vi "UHR-Fleezers Control (host) - 10.8MV_trial.vi"() -> ()   [LabVIEW 2010] (continued)
      n270 = call <vilib>:"Application Directory.vi"() -> ("Application Directory"=w928:path)
      n271 = Build Path(base path=w928, name or relative path="_trap_screen_positions") -> (appended path=w936:path)
      n272 = Open/Create/Replace File(file path (use dialog)=w936, operation (0:open)=T25."open or create", access (0:read/write)=enum16{"read/write", "read-only", "write-only"}."read/write") -> (refnum out=w938:refnum<file>)  [unwired: 3 in, 2 out]
      n273 = local read "Trap Sets"() -> (w930:u32)
      n274 = for "Load trap positions on video screen from file." {
        N: w930 -> [_]
        tunnel: [w956] -> w931
        tunnel: w938 -> [w955]
        tunnel: [w952] -> w927 mode=indexing
        w954 = 4
        n275 = for {
          N: w954 -> [_]
          tunnel: [w960] -> w956
          tunnel: w955 -> [w959]
          tunnel: w954 -> [w958]
          tunnel: [w957] -> w953 mode=indexing
          n276 = Read from Binary File(5:w958, 11:w959) -> (2:w957:i32, 3:w960:refnum<file>)  [unwired: 4 in, 2 out]
        }
        n277 = Array To Cluster(array=w953) -> (cluster=w952:T29)
      }
      n278 = node-c288() -> (w951:T26)  [unwired: 4 in]
      n279 = timed-loop "acquire video and stage position" {
        timing: w951 -> [_]
        timing-out: [_] -> w950
        tunnel: w943 -> [w979]
        tunnel: w942 -> [w978]
        tunnel: w941 -> [w977]
        tunnel: [w976] -> w923
        tunnel: [w973] -> w924
        tunnel: [w974] -> w922
        tunnel: w949 -> [_]
        shift-right: [w970] -> w940
        shift-left: w927 -> [w971]
        tunnel: w930 -> [w968]
        stop <- w975 stop-if-true
        n280 = node-c288() -> ()  [unwired: 1 in, 1 out]
        n281 = event shown="[2] \"Primary Video Display\": Mouse Down" {
          selector: _ -> [_ _ _ _]
          dyn-events: _ -> [_ _ _ _]
          timeout: 10 -> [_ _ _ _]
          tunnel: w979 -> [w990 w1005 w1014 w1033]
          tunnel: w978 -> [w989 w1007 w1012 w1035]
          tunnel: w977 -> [w988 w1006 w1013 w1034]
          tunnel: [w987 w1005 w1014 w1033] -> w976
          tunnel: [w980 w1009 FALSE FALSE] -> w975
          tunnel: [w984 w1007 w1012 w1035] -> w974
          tunnel: [w983 w1006 w1013 w1034] -> w973
          tunnel: "radius" -> [_ _ w1019 _]
          tunnel: w971 -> [w981 w1008 w1017 _]
          tunnel: [w981 w1008 w1018 cluster{i32, i32, i32, i32}[] []] -> w970
          tunnel: w968 -> [_ _ w1010 _]
          event Timeout {
            n282 = event-data() -> ()  [unwired: 1 in, 2 out]
            n283 = call <vilib>:"IMAQ Grab Acquire.vi"("error in (no error)"=w989, "Image In"=w988, "IMAQ Session In"=w990) -> ("error out"=w985:errorcluster, "Image Out"=w986:T2, "IMAQ Session Out"=w987:refnum<k11>)  [unwired: 5 in, 1 out]
            n284 = case shown="True" "trap\nmarkers?" {
              tunnel: w981 -> [_ w998]
              tunnel: w986 -> [w992 w997]
              tunnel: w985 -> [w991 w996]
              tunnel: [w991 w995] -> w984
              tunnel: [w992 w993] -> w983
              frame False {
              }
              frame True {
                n285 = for {
                  tunnel: w998 -> [w1004] mode=indexing
                  shift-right: [w1002] -> w993
                  shift-left: w997 -> [w1003]
                  tunnel: w996 -> [w1001]
                  tunnel: [w1000] -> w995
                  tunnel: u32 16711680 ("Color") -> [w999]
                  n286 = call "IMAQ Overlay Oval"("Color"=w999, "error in (no error)"=w1001, "Bounding Rectangle"=w1004, "Image"=w1003) -> ("error out"=w1000:errorcluster, "Image Out"=w1002:T2)  [unwired: 6 in]
                }
              }
            }
            "Primary Video Display" <- w983
            n287 = Unbundle By Name(w985) -> ("status"=w980:bool)
          }
          event "Stop All": Value Change {
            n288 = event-data() -> ()  [unwired: 1 in, 5 out]
            n289 = local read "Stop All"() -> (w1009:bool)
          }
          event "Primary Video Display": Mouse Down {
            n290 = event-data() -> ()  [unwired: 1 in, 7 out]
            n291 = Array Size(array=w1017) -> (size(s)=w1016:i32)
            n292 = Less?(x=w1016, y=w1010) -> (x < y?=w1015:bool)
            n293 = case shown="True" w1015 {
              tunnel: w1019 -> [_ w1029]
              tunnel: w1017 -> [w1020 w1023]
              tunnel: [w1020 w1022] -> w1018
              frame False {
              }
              frame True {
                n294 = property on="Primary Video Display" class="ImageControl"() -> ("Last Mouse Position"=w1021:cluster{"X":i32, "Y":i32})  [unwired: 2 in, 2 out]
                n295 = Unbundle By Name(w1021) -> ("X"=w1031:i32, "Y"=w1030:i32)
                n296 = Add(x=w1030, y=w1029) -> (x+y=w1027:i32)
                n297 = Subtract(x=w1030, y=w1029) -> (x-y=w1025:i32)
                n298 = Add(x=w1031, y=w1029) -> (x+y=w1026:i32)
                n299 = Subtract(x=w1031, y=w1029) -> (x-y=w1028:i32)
                n300 = Bundle(w1028, w1027, w1026, w1025) -> (w1024:cluster{i32, i32, i32, i32})  [unwired: 1 in]
                n301 = Build Array (concatenate)(w1023, w1024) -> (w1022:T30)
              }
            }
          }
          event "clear markers": Value Change {
            n302 = event-data() -> ()  [unwired: 1 in, 5 out]
          }
        }
        n303 = node-c288() -> ()  [unwired: 1 in, 1 out]
      }
      n304 = node-c288(w950) -> ()  [unwired: 1 out]
      n305 = Set File Position(offset (in bytes) (0)=i64 0, refnum=w931, from (0:start)=enum16{"start", "end", "current"}."start") -> (refnum out=w932:refnum<file>)  [unwired: 1 in, 1 out]
      n306 = for "Write trap positions to file so they can be remembered\nwhen program is removed from memory" {
        tunnel: w940 -> [w964] mode=indexing
        tunnel: [w962] -> w939
        tunnel: w932 -> [w961]
        n307 = Cluster To Array(cluster=w964) -> (array=w963:i32[])
        n308 = for {
          tunnel: w963 -> [w967] mode=indexing
          tunnel: [w966] -> w962
          tunnel: w961 -> [w965]
          n309 = Write to Binary File(file (use dialog)=w965, data=w967) -> (refnum out=w966:refnum<file>)  [unwired: 4 in, 2 out]
        }
      }
      n310 = Close File(refnum=w939) -> ()  [unwired: 1 in, 2 out]
      n311 = call "IMAQ Dispose"("Image"=w924, "error in (no error)"=w922) -> ("error out"=w921:errorcluster)  [unwired: 4 in]
      n312 = call <vilib>:"IMAQ Stop.vi"("error in (no error)"=w921, "IMAQ Session In"=w923) -> ("error out"=w925:errorcluster, "IMAQ Session Out"=w926:refnum<k11>)  [unwired: 8 in]
      n313 = call <vilib>:"IMAQ Close.vi"("error in (no error)"=w925, "IMAQ Session In"=w926) -> ()  [unwired: 9 in, 1 out]
    }
    frame Enabled {
    }
  }
  n314 = node-c288(2 ("Processor")) -> (w15:T26)  [unwired: 3 in]
  n315 = node-c288() -> (w69:T26)  [unwired: 4 in]
  n316 = disable-structure shown="Enabled" {
    disable-tunnel: [w1042 _] -> w35
    disable-tunnel: w24 -> [w1041 _]
    frame Enabled {
      n317 = node-c288() -> (w1044:T26)  [unwired: 4 out]
      n318 = timed-loop "Rough control of MCL mirror stage (debugging)" {
        tunnel: w1041 -> [w1047]
        tunnel: [w1046] -> w1042
        timing: w1044 -> [_]
        timing-out: [_] -> w1043
        stop <- w1046 stop-if-true
        n319 = node-c288() -> ()  [unwired: 2 out]
        n320 = case shown="1" "MCL Mode" {
          tunnel: w1047 -> [_ w1050 w1154]
          frame 0, Default {
            # "manual positioning"
          }
          frame 1 {
            # "sinusoidal wave"
            n321 = node-c288() -> (w1052:T26)  [unwired: 4 out]
            n322 = timed-loop "Oscillate MCL mirror" {
              timing: w1052 -> [_]
              timing-out: [_] -> w1051
              tunnel: w1050 -> [w1091]
              i -> [w1090]
              stop <- w1053 stop-if-true
              n323 = node-c288() -> (w1089:i64)  [unwired: 1 out]
              n324 = Multiply(x="AO1", y=32767.0) -> (x*y=w1085:dbl)
              n325 = Multiply(x="AO2", y=32767.0) -> (x*y=w1080:dbl)
              n326 = Divide(x=w1085, y=10.0) -> (x/y=w1086:dbl)
              n327 = Divide(x=w1080, y=10.0) -> (x/y=w1081:dbl)
              n328 = To Word Integer(number=w1086) -> (16bit integer=w1078:i16)
              n329 = To Word Integer(number=w1081) -> (16bit integer=w1077:i16)
              n330 = Divide(x=w1089, y=i64 1000) -> (x/y=w1060:dbl)
              n331 = Multiply(x=w1060, y=w1090) -> (x*y=w1071:dbl)
              n332 = Multiply(x="Osc. freq. (Hz) 2", y=6.283185307179586) -> (x*y=w1072:dbl)
              n333 = Multiply(x=w1072, y=w1071) -> (x*y=w1070:dbl)
              n334 = Sine(x=w1070) -> (sin(x)=w1069:dbl)
              n335 = Multiply(x=w1069, y="Osc. amp. (V)") -> (x*y=w1067:dbl)
              n336 = Add(x=w1067, y="Osc. center (V)") -> (x+y=w1065:dbl)
              n337 = Divide(x=w1065, y=10.0) -> (x/y=w1063:dbl)
              n338 = Multiply(x=w1063, y=32767.0) -> (x*y=w1058:dbl)
              n339 = Select(t=w1058, s="Scan axis", f=w1078) -> (s? t:f=w1076:dbl)
              n340 = Select(t=w1077, s="Scan axis", f=w1058) -> (s? t:f=w1075:dbl)
              n341 = local read "MCL Mode"() -> (w1057:u16)
              n342 = Not Equal?(x=w1057, y=u16 1) -> (x != y?=w1054:bool)
              n343 = local read "Stop All"() -> (w1055:bool)
              n344 = xnode "Read/Write Control"("FPGA VI Reference In"=w1091, "AO1"=w1076, "AO2"=w1075) -> ()  [unwired: 1 in, 2 out]
              n345 = Compound Arithmetic op=OR(w1055, w1054) -> (w1053:bool)
              n346 = node-c288() -> ()  [unwired: 2 out]
            }
            n347 = node-c288(w1051) -> ()  [unwired: 1 out]
          }
          frame 2 {
            # "linear scan"
            n348 = case shown="True" "Start Scan" {
              tunnel: w1154 -> [_ w1166]
              frame False {
              }
              frame True {
                n349 = Subtract(x="End (V)", y="Begin (V)") -> (x-y=w1162:dbl)
                n350 = Decrement(x="N Points") -> (x-1=w1161:dbl)
                n351 = Divide(x=w1162, y=w1161) -> (x/y=w1159:dbl)
                n352 = for {
                  N: "N Points" -> [_]
                  tunnel: "Begin (V)" -> [w1179]
                  tunnel: w1166 -> [w1171]
                  tunnel: [w1170] -> w1165 mode=indexing
                  tunnel: w1159 -> [w1169]
                  tunnel: [w1167] -> w1158 mode=indexing
                  i -> [w1178]
                  n353 = Multiply(x=w1169, y=w1178) -> (x*y=w1177:dbl)
                  n354 = Add(x=w1179, y=w1177) -> (x+y=w1174:dbl)
                  n355 = local read "Scan axis"() -> (w1168:bool)
                  n356 = local read "AO1"() -> (w1176:dbl)
                  n357 = local read "AO2"() -> (w1175:dbl)
                  n358 = Select(t=w1174, s=w1168, f=w1176) -> (s? t:f=w1173:dbl)
                  n359 = Select(t=w1175, s=w1168, f=w1174) -> (s? t:f=w1172:dbl)
                  n360 = flat-sequence {
                    tunnel: w1173 -> [w1183]
                    tunnel: w1172 -> [w1182]
                    tunnel: w1171 -> [w1180]
                    tunnel: [w1250] -> w1170
                    tunnel: [w1249] -> w1167
                    frame #0 {
                      w1186 = 10.0 ("y")
                      w1181 = 32767.0 ("y")
                      n361 = Multiply(x=w1183, y=w1181) -> (x*y=w1189:dbl)
                      n362 = Multiply(x=w1182, y=w1181) -> (x*y=w1187:dbl)
                      n363 = Divide(x=w1189, y=w1186) -> (x/y=w1190:dbl)
                      n364 = Divide(x=w1187, y=w1186) -> (x/y=w1188:dbl)
                      n365 = To Word Integer(number=w1190) -> (16bit integer=w1184:i16)
                      n366 = To Word Integer(number=w1188) -> (16bit integer=w1185:i16)
                      n367 = xnode "Read/Write Control"("FPGA VI Reference In"=w1180, "AO1"=w1184, "AO2"=w1185) -> ()  [unwired: 1 in, 2 out]
                    }
                    frame #1 {
                      n368 = Wait (ms)(milliseconds to wait="DAQ Delay (ms)") -> ()  [unwired: 1 out]
                    }
                    frame #2 {
                      n369 = local read "Slow mean"() -> (w1250:dbl)
                      n370 = local read "Sigma"() -> (w1249:dbl)
                    }
                  }
                }
                n371 = Bundle("Begin (V)"="Begin (V)", w1159, w1165) -> (→"MCL Scan":cluster{"Begin (V)":dbl, dbl, dbl[]})  [unwired: 1 out]
                n372 = Bundle("Begin (V)"="Begin (V)", w1159, w1158) -> (→"MCL Scan 2":cluster{"Begin (V)":dbl, dbl, dbl[]})  [unwired: 1 out]
              }
            }
          }
        }
        n373 = local read "Stop All"() -> (w1046:bool)
        n374 = node-c288() -> ()  [unwired: 2 out]
      }
      n375 = node-c288(w1043) -> ()  [unwired: 1 out]
    }
    frame Disabled {
    }
  }
  n376 = timed-loop "Control parameters (event loop)" {
    tunnel: w24 -> [w1256]
    shift-right: [w1255] -> _
    shift-left: errorcluster {"status"=FALSE, "code"=0, "source"=""} ("error out") -> [w1254]
    tunnel: [w1253] -> w37
    timing: w15 -> [_]
    timing-out: [_] -> w14
    stop <- w1253 stop-if-true
    n377 = node-c288() -> ()  [unwired: 1 in, 1 out]
    n378 = event shown="[6] \"BD 1 Frequency 1 (MHz)\", \"BD 1 Frequency 2 (MHz)\", \"BD 1 Frequency 3 (MHz)\", \"BD 2 Frequency 1 (MHz)\", \"BD 2 Frequency 2 (MHz)\", \"BD 2 Frequency 3 (MHz)\", \"Trap Delta (MHz)\": Value Change" {
      selector: _ -> [_ _ _ _ _ _ _ _ _ _ _ _ _ _ _ _ _ _ _ _ _ _ _ _ _ _ _ _ _ _ _ _ _ _ _ _ _ _ _ _ _ _ _ _ _ _ _ _ _ _ _ _ _ _ _]
      dyn-events: _ -> [_ _ _ _ _ _ _ _ _ _ _ _ _ _ _ _ _ _ _ _ _ _ _ _ _ _ _ _ _ _ _ _ _ _ _ _ _ _ _ _ _ _ _ _ _ _ _ _ _ _ _ _ _ _ _]
      timeout: _ -> [_ _ _ _ _ _ _ _ _ _ _ _ _ _ _ _ _ _ _ _ _ _ _ _ _ _ _ _ _ _ _ _ _ _ _ _ _ _ _ _ _ _ _ _ _ _ _ _ _ _ _ _ _ _ _]
      tunnel: w1256 -> [w1294 _ _ _ w1416 _ w1513 _ w1577 _ _ _ w1772 _ _ w1874 w2018 w2082 w2157 w2311 w2388 w2519 w2615 w2701 w2787 w2873 w2959 w3045 w3138 w3302 w3513 _ w3658 w3795 _ w4002 w4044 w4092 w4171 w4213 _ w4259 _ _ _ _ w4450 _ w4543 w4584 w4631 w4819 w4868 _ w4930]
      tunnel: [w1293 _ _ _ w1406 _ w1512 _ w1540 _ w1737 _ w1751 _ _ w1873 w2014 w2079 w2154 w2310 w2386 w2518 w2609 w2695 w2781 w2867 w2953 w3039 w3136 w3301 w3511 _ w3656 w3793 _ w4000 w4042 w4082 w4169 w4211 _ w4257 _ _ _ _ w4448 _ _ _ _ _ _ _ _] -> w1255
      tunnel: w1254 -> [w1292 _ _ _ w1415 _ w1511 _ w1572 _ w1737 _ w1771 _ _ w1872 w2013 w2078 w2153 w2309 w2387 w2517 w2614 w2700 w2786 w2872 w2958 w3044 w3137 w3300 w3512 _ w3657 w3794 _ w4001 w4043 w4091 w4170 w4212 _ w4258 _ _ _ _ w4449 _ w4542 w4583 w4630 w4818 w4867 _ w4929]
      tunnel: [_ _ _ _ _ _ _ _ _ _ w1736 _ _ _ _ _ _ _ _ _ _ _ _ _ _ _ _ _ _ _ _ _ _ _ _ _ _ _ _ _ _ _ _ _ _ _ _ _ _ _ _ _ _ _ _] -> w1253
      tunnel: [_ _ _ _ _ _ _ "Round T1 X" _ _ _ _ _ _ _ _ _ _ _ _ _ _ _ _ _ _ _ _ _ _ _ _ _ _ _ _ _ _ _ _ _ _ _ _ _ _ _ _ _ _ _ _ _ _ _] -> _
      tunnel: [_ _ _ "Adjust Scale\nto Mean" _ _ _ _ _ _ _ _ _ _ _ _ _ _ _ _ _ _ _ _ _ _ _ _ _ _ _ _ _ _ _ _ _ _ _ _ _ _ _ _ _ _ _ _ _ _ _ _ "Set SP to Reading" _ _] -> _
      tunnel: [_ _ _ _ _ _ _ _ _ "Round T2 X" _ "Delayed Interlace Start" _ _ _ _ _ _ _ _ _ _ _ _ _ _ _ _ _ _ _ _ _ _ _ _ _ _ _ _ _ _ _ _ _ _ _ _ _ _ _ _ _ _ _] -> _
      event "AI Count (ticks)", "Sets to FIFO (Traps)", "Save ave N", "FPGA Ave.", "# Samples/channel", "N sets to save": Value Change {
        # "So that if 'Save ave N' is updated, the AOD scanning code updates too."
        n379 = event-data() -> ()  [unwired: 6 out]
        n380 = local read "AI Count (ticks)"() -> (w1274:u32)
        n381 = Boolean To (0,1)(Boolean="Sets to FIFO (Traps)") -> (0, 1=w1284:cluster{"Set 1":i16, "Set 2":i16, "Set 3":i16})
        n382 = xnode "Read/Write Control"("FPGA VI Reference In"=w1294, "error in"=w1292, "ai count"=w1274, "AI1 Sets to FIFO"="Sets to FIFO (Traps)", "N of AI1 Int Acq Sets"="N Acq Sets (Traps + Fl.)") -> ("error out"=w1293:errorcluster)  [unwired: 1 out]
        n383 = Cluster To Array(cluster=w1284) -> (array=w1283:i16[])
        n384 = To Unsigned Long Integer(number=w1283) -> (unsigned 32bit integer=w1263:u32[])
        n385 = local read "Scan steps (AOD)"() -> (w1285:u64)
        n386 = Multiply(x=w1274, y="N Acq Sets (Traps + Fl.)") -> (x*y=w1272:u32)
        n387 = Divide(x=40000000.0, y=w1274) -> (x/y=w1266:dbl)
        "AI rate (Hz)" <- w1266
        "Ave. Rate (Hz)" <- w1266
        n388 = Add Array Elements(numeric array=w1263) -> (sum=w1275:u32)
        "Trap Sets" <- w1275
        n389 = Reciprocal(x=w1266) -> (1/x=→"Ave. Period (s)":dbl)
        n390 = property on="Scan steps (AOD)" class="DigNum (strict)"("Val(Sgnl)"=w1285) -> ()  [unwired: 2 in, 2 out]
        n391 = Divide(x=w1266, y="N Acq Sets (Traps + Fl.)") -> (x/y=w1289:dbl)
        "Data Rate (Hz)" <- w1289
        n392 = Reciprocal(x=w1289) -> (1/x=→"Data Period (s)":dbl)
        n393 = local read "Save ave N"() -> (w1288:dbl)
        n394 = Divide(x=w1289, y=w1288) -> (x/y=w1287:dbl)
        "Save Data Rate (Hz)" <- w1287
        n395 = Reciprocal(x=w1287) -> (1/x=→"Save Data Period (s)":dbl)
        n396 = Multiply(x=w1272, y="# Samples/trap") -> (x*y=w1270:u32)
        "Counts/DMA" <- w1270
        n397 = property on="Trap Disp. Downsample" class="DigNum (strict)"("Maximum"="# Samples/trap") -> ()  [unwired: 2 in, 2 out]
        n398 = Multiply(x=w1275, y="# Samples/trap") -> (x*y=w1264:u32)
        "# Samples/channel" <- w1264
        n399 = Multiply(x=w1264, y=u32 8) -> (x*y=→"Trap AI Elements/DMA read":u32)
        n400 = local read "APD Int. Count"() -> (w1271:u32)
        n401 = Multiply(x=w1264, y=u32 3) -> (x*y=→"Trap Pos Elements/DMA read":u32)
        n402 = Divide(x=w1270, y=w1271) -> (x/y=w1261:dbl)
        "APD Samples/FIFO Acq." <- w1261
        n403 = Divide(x=w1270, y=40000000.0) -> (x/y=w1268:dbl)
        "DMA Update Period (s)" <- w1268
        n404 = Multiply(x=2.0, y=w1261) -> (x*y=→"APD Elements/DMA read":dbl)
        n405 = property on="APD Disp. Downsample" class="DigNum (strict)"("Maximum"=w1261) -> ()  [unwired: 2 in, 2 out]
        n406 = local read "N sets to save"() -> (w1281:u32)
        n407 = Multiply(x=w1268, y=w1281) -> (x*y=→"Total Time (s)":dbl)
        "FPGA Averaging" <- FALSE ("FPGA Averaging")
      }
      event "Rescale on Mean": Value Change {
        n408 = event-data() -> ()  [unwired: 7 out]
        n409 = And(x=FALSE, y="Rescale on Mean") -> (x .and. y?=w1381:bool)
        n410 = local write "Rescale on Mean"(w1381) -> ()
        n411 = local read "Bead Mean (nm)"() -> (w1386:dbl)
        n412 = Add(x="Amplitude (nm)", y=w1386) -> (x+y=w1384:dbl)
        n413 = Subtract(x=w1386, y="Amplitude (nm)") -> (x-y=w1383:dbl)
        n414 = property on="Bead Separation" class="WFChart (strict)"("YScale.Minimum"=w1383) -> ()  [unwired: 2 in, 2 out]
        n415 = property on="Bead Separation" class="WFChart (strict)"("YScale.Maximum"=w1384) -> ()  [unwired: 2 in, 2 out]
      }
      event "Detector Type": Value Change {
        n416 = event-data() -> ()  [unwired: 7 out]
        n417 = local read "AI labels"() -> (w1387:string[])
        n418 = property on="High Res. Display" class="Ring (strict)"("Strings []"=w1387) -> ()  [unwired: 2 in, 2 out]
        n419 = Build Array (concatenate)(w1387, "none") -> (w1388:string[])
        n420 = property on="FFT 1 Choice 1" class="Ring (strict)"("Strings []"=w1388) -> ()  [unwired: 2 in, 2 out]
        n421 = property on="FFT 1 Choice 2" class="Ring (strict)"("Strings []"=w1388) -> ()  [unwired: 2 in, 2 out]
        n422 = property on="FFT 2 Choice 1" class="Ring (strict)"("Strings []"=w1388) -> ()  [unwired: 2 in, 2 out]
        n423 = property on="FFT 2 Choice 2" class="Ring (strict)"("Strings []"=w1388) -> ()  [unwired: 2 in, 2 out]
        n424 = Bundle("APD 1", "APD 2") -> (w1391:cluster{string, string})  [unwired: 1 out]
        n425 = Cluster To Array(cluster=w1391) -> (array=w1389:string[])
        n426 = Build Array (concatenate)(w1389, w1388) -> (w1393:string[])
        n427 = Array Size(array=w1393) -> (size(s)=w1394:i32)
        n428 = property on="Signals to Plot" class="LstBox (strict)"("Item Names"=w1393) -> ()  [unwired: 2 in, 2 out]
        n429 = property on="Signals to Plot" class="LstBox (strict)"("Number of Rows"=w1394) -> ()  [unwired: 2 in, 2 out]
        n430 = property on="All Signals" class="WFChart (strict)"("LegNumRows"=w1394) -> ()  [unwired: 2 in, 2 out]
      }
      event "Adjust Scale\nto Mean": Value Change {
        n431 = event-data() -> ()  [unwired: 7 out]
        n432 = local read "APD 1 Rate (Hz)"() -> (w1403:dbl)
        n433 = Multiply(x=1000.0, y="Above (kHz)") -> (x*y=w1401:dbl)
        n434 = Multiply(x=1000.0, y="Below (kHz)") -> (x*y=w1399:dbl)
        n435 = Add(x=w1401, y=w1403) -> (x+y=w1396:dbl)
        n436 = Subtract(x=w1403, y=w1399) -> (x-y=w1397:dbl)
        n437 = property on="APD Chart" class="WFChart (strict)"("YScale.Minimum"=w1397) -> ()  [unwired: 2 in, 2 out]
        n438 = property on="APD Chart" class="WFChart (strict)"("YScale.Maximum"=w1396) -> ()  [unwired: 2 in, 2 out]
      }
      event "Phase adj. (AI1)", "+ phase (AI1)", "- phase (AI1)": Value Change {
        n439 = event-data() -> ()  [unwired: 7 out]
        n440 = Negate(x="Phase adj. (AI1)") -> (-x=w1413:i16)
        n441 = Select(t=w1413, s="- phase (AI1)", f="Phase adj. (AI1)") -> (s? t:f=w1412:i16)
        n442 = xnode "Read/Write Control"("FPGA VI Reference In"=w1416, "error in"=w1415, "Phase count adjustment"=w1412) -> ("FPGA VI Reference Out"=w1411:T19, "error out"=w1410:errorcluster)
        n443 = Or(x="- phase (AI1)", y="+ phase (AI1)") -> (x .or. y?=w1407:bool)
        n444 = xnode "Read/Write Control"("FPGA VI Reference In"=w1411, "error in"=w1410, "+ phase"=w1407) -> ("error out"=w1406:errorcluster)  [unwired: 1 out]
      }
      event "Signals to Plot": Double Click {
        w1494 = u32 9868950 ("Color Box")
        n445 = event-data() -> ("Row"=w1496:i32)  [unwired: 9 out]
        n446 = property on="All Signals" class="WFChart (strict)"("Active Plot"=w1496) -> (error out=w1507:errorcluster)  [unwired: 2 in, 1 out]
        n447 = property on="All Signals" class="WFChart (strict)" props=["Plot", "Visible?", "Plot", "Plot Color"](error in=w1507) -> (error out=w1506:errorcluster, "Plot.Visible?"=w1505:bool)  [unwired: 1 in, 2 out]
        n448 = Select(t=FALSE ("Plot.Visible"), s=w1505, f=TRUE ("Plot.Visible")) -> (s? t:f=w1500:bool)
        n449 = property on="All Signals" class="WFChart (strict)"(error in=w1506, "Plot.Visible?"=w1500) -> (error out=w1502:errorcluster)  [unwired: 1 in, 1 out]
        n450 = property on="All Signals" class="WFChart (strict)"(error in=w1502) -> (error out=w1497:errorcluster, "Plot.Plot Color"=w1501:u32)  [unwired: 1 in, 1 out]
        n451 = property on="Signals to Plot" class="LstBox (strict)"(error in=w1497, "Active Row"=w1496) -> (error out=w1495:errorcluster)  [unwired: 1 in, 1 out]
        n452 = Select(t=w1501, s=w1500, f=u32 0) -> (s? t:f=w1498:u32)
        n453 = property on="Signals to Plot" class="LstBox (strict)"(error in=w1495, "CellFontColor"=w1498, "SelColor"=w1494, "CellBG"=w1494, "CellFontSize"=u32 20 ("Active Row:Cell Font:Size"), "CellFontBold"=TRUE ("Active Row:Cell Font:Bold")) -> ()  [unwired: 1 in, 2 out]
      }
      event "BD 1 Frequency 1 (MHz)", "BD 1 Frequency 2 (MHz)", "BD 1 Frequency 3 (MHz)", "BD 2 Frequency 1 (MHz)", "BD 2 Frequency 2 (MHz)", "BD 2 Frequency 3 (MHz)", "Trap Delta (MHz)": Value Change {
        # "anytime one of the frequencies is changed, write it to the RF board UNLESS Set 2 is being oscillated. The oscillation\nscript writes the frequencies to the RF board."
        n454 = event-data() -> ("CtlRef"=w1510:refnum<vi>)  [unwired: 6 out]
        n455 = control-ref of="Trap Delta (MHz)"() -> (w1509:refnum<vi>)
        n456 = Equal?(x=w1509, y=w1510) -> (x = y?=w1508:bool)
        n457 = case shown="False" "Oscillate Set 2" {
          tunnel: w1513 -> [w1533 _]
          tunnel: [w1532 w1536] -> w1512
          tunnel: w1511 -> [w1531 w1536]
          tunnel: w1508 -> [w1517 _]
          frame False {
            n458 = local read "BD 1 Frequency 1 (MHz)"() -> (w1515:dbl)
            n459 = local read "BD 1 Frequency 2 (MHz)"() -> (w1519:dbl)
            n460 = Add(x=w1515, y="Trap Delta (MHz)") -> (x+y=w1518:dbl)
            n461 = Select(t=w1518, s=w1517, f=w1519) -> (s? t:f=w1516:dbl)
            n462 = local read "Y RF Frequency Limits (MHz)"() -> (w1521:T16)
            n463 = local read "X RF Frequency Limits (MHz)"() -> (w1522:T16)
            n464 = local read "BD 1 Frequency 3 (MHz)"() -> (w1534:dbl)
            n465 = local write "BD 1 Frequency 2 (MHz)"(w1516) -> ()
            n466 = local read "BD 2 Frequency 1 (MHz)"() -> (w1525:dbl)
            n467 = local read "BD 2 Frequency 2 (MHz)"() -> (w1524:dbl)
            n468 = local read "BD 2 Frequency 3 (MHz)"() -> (w1535:dbl)
            n469 = call "set RF board frequency - interlace.vi"("Board 2 Frequency Limits"=w1521, "Board 1 Frequency Limits"=w1522, "error in"=w1531, "FPGA VI Reference In"=w1533, "Board 2 Frequency 3 (MHz)"=w1535, "Board 1 Frequency 3 (MHz)"=w1534, "Board 2 Frequency 2 (MHz)"=w1524, "Board 2 Frequency 1 (MHz)"=w1525, "Board 1 Frequency 2 (MHz)"=w1516, "Board 1 Frequency 1  (MHz)"=w1515) -> ("error out"=w1532:errorcluster)  [unwired: 1 out]
            n470 = Subtract(x=w1525, y=w1524) -> (x-y=w1529:dbl)
            n471 = Subtract(x=w1516, y=w1515) -> (x-y=w1530:dbl)
            n472 = Square(x=w1529) -> (x^2=w1527:dbl)
            n473 = Square(x=w1530) -> (x^2=w1528:dbl)
            n474 = Add(x=w1528, y=w1527) -> (x+y=w1526:dbl)
            n475 = Square Root(x=w1526) -> (sqrt(x)=w1523:dbl)
            n476 = local write "Trap Delta (MHz)"(w1523) -> ()
            n477 = property on="Initial delta (MHz)" class="DigNum (strict)"("Val(Sgnl)"=w1523) -> ()  [unwired: 2 in, 2 out]
          }
          frame True {
          }
        }
      }
      event "Round T1 X": Value Change {
        n478 = event-data() -> ()  [unwired: 7 out]
        n479 = local read "BD 1 Frequency 1 (MHz)"() -> (w1539:dbl)
        n480 = Round To Nearest(number=w1539) -> (nearest integer value=w1538:dbl)
        n481 = property on="BD 1 Frequency 1 (MHz)" class="DigNum (strict)"("Val(Sgnl)"=w1538) -> ()  [unwired: 2 in, 2 out]
      }
      event "Restart RF": Value Change {
        n482 = event-data() -> ()  [unwired: 7 out]
        n483 = xnode "Read/Write Control"("FPGA VI Reference In"=w1577, "error in"=w1572, "FPGA Controls  RF Box"=FALSE) -> ("FPGA VI Reference Out"=w1576:T19, "error out"=w1571:errorcluster)
        n484 = local read "Y RF Amplitude Limits (%)"() -> (w1552:T16)
        n485 = local read "X RF Amplitude Limits (%)"() -> (w1553:T16)
        n486 = local read "X RF Frequency Limits (MHz)"() -> (w1555:T16)
        n487 = local read "Y RF Frequency Limits (MHz)"() -> (w1554:T16)
        n488 = xnode "Read/Write Control"("FPGA VI Reference In"=w1576, "error in"=w1571, "Direct RF Box  Communication"=TRUE) -> ("FPGA VI Reference Out"=w1575:T19, "error out"=w1570:errorcluster)
        n489 = local read "BD 2 Frequency 3 (MHz)"() -> (w1562:dbl)
        n490 = local read "BD 2 Frequency 2 (MHz)"() -> (w1563:dbl)
        n491 = local read "BD 1 Frequency 3 (MHz)"() -> (w1566:dbl)
        n492 = local read "BD 1 Frequency 1 (MHz)"() -> (w1567:dbl)
        n493 = local read "BD 2 Frequency 1 (MHz)"() -> (w1564:dbl)
        n494 = local read "BD 1 Frequency 2 (MHz)"() -> (w1565:dbl)
        n495 = call "Initialize RF boards - interlace 3.vi"("error in"=w1570, "FPGA VI Reference In"=w1575) -> ("error out"=w1569:errorcluster, "FPGA VI Reference Out"=w1574:T19)
        n496 = local read "BD 2 Amplitude 2 (%)"() -> (w1557:dbl)
        n497 = local read "BD 2 Amplitude 1 (%)"() -> (w1558:dbl)
        n498 = local read "BD 2 Amplitude 3 (%)"() -> (w1556:dbl)
        n499 = local read "BD 1 Amplitude 3 (%)"() -> (w1561:dbl)
        n500 = local read "BD 1 Amplitude 1 (%)"() -> (w1560:dbl)
        n501 = local read "BD 1 Amplitude 2 (%)"() -> (w1559:dbl)
        n502 = call "set RF board frequency - interlace.vi"("Board 2 Frequency Limits"=w1554, "Board 1 Frequency Limits"=w1555, "error in"=w1569, "FPGA VI Reference In"=w1574, "Board 2 Frequency 3 (MHz)"=w1562, "Board 1 Frequency 3 (MHz)"=w1566, "Board 2 Frequency 2 (MHz)"=w1563, "Board 2 Frequency 1 (MHz)"=w1564, "Board 1 Frequency 2 (MHz)"=w1565, "Board 1 Frequency 1  (MHz)"=w1567) -> ("error out"=w1568:errorcluster, "FPGA VI Reference Out"=w1573:T19)
        n503 = call "set RF board amplitude - interlace.vi"("Board 2 Amplitude Limits"=w1552, "Board 1 Amplitude Limits"=w1553, "error in"=w1568, "FPGA VI Reference In"=w1573, "Board 2 Amplitude 3 (%)"=w1556, "Board 1 Amplitude 3 (%)"=w1561, "Board 2 Amplitude 2 (%)"=w1557, "Board 2 Amplitude 1 (%)"=w1558, "Board 1 Amplitude 2 (%)"=w1559, "Board 1 Amplitude 1 (%)"=w1560) -> ("error out"=w1545:errorcluster, "FPGA VI Reference Out"=w1549:T19)
        n504 = xnode "Read/Write Control"("FPGA VI Reference In"=w1549, "error in"=w1545, "Direct RF Box  Communication"=FALSE) -> ("FPGA VI Reference Out"=w1548:T19, "error out"=w1547:errorcluster)
        n505 = flat-sequence {
          tunnel: w1547 -> [w1578]
          tunnel: [w1578] -> w1546
          frame #0 {
            n506 = Wait (ms)(milliseconds to wait=u32 50) -> ()  [unwired: 1 out]
          }
        }
        n507 = xnode "Read/Write Control"("FPGA VI Reference In"=w1548, "error in"=w1546, "FPGA Controls  RF Box"=TRUE) -> ("error out"=w1541:errorcluster)  [unwired: 1 out]
        n508 = property on="Restart RF" class="Bool (strict)"(error in=w1541, "Value"=FALSE ("Restart RF")) -> (error out=w1540:errorcluster)  [unwired: 1 in, 1 out]
      }
      event "Round T2 X": Value Change {
        n509 = event-data() -> ()  [unwired: 7 out]
        n510 = local read "BD 1 Frequency 2 (MHz)"() -> (w1733:dbl)
        n511 = Round To Nearest(number=w1733) -> (nearest integer value=w1732:dbl)
        n512 = property on="BD 1 Frequency 2 (MHz)" class="DigNum (strict)"("Val(Sgnl)"=w1732) -> ()  [unwired: 2 in, 2 out]
      }
      event "Stop All": Value Change {
        n513 = event-data() -> ()  [unwired: 7 out]
        n514 = call "hamilton_controller.vi"("action"=T22."DISCONNECT") -> ()  [unwired: 10 in, 1 out]
        n515 = local read "Stop All"() -> (w1736:bool)
      }
      event "Delayed Interlace Start": Value Change {
        n516 = event-data() -> ()  [unwired: 7 out]
        n517 = flat-sequence {
          frame #0 {
            n518 = Multiply(x="Delay to Interlace (s)", y=1000.0) -> (x*y=w1739:dbl)
            n519 = Wait (ms)(milliseconds to wait=w1739) -> ()  [unwired: 1 out]
          }
          frame #1 {
            n520 = property on="Green laser mode" class="RadioBtnsControl (strict)"("Val(Sgnl)"=enum32{"Laser ON", "Laser OFF", "Interlace"}."Interlace" ("Value (Signaling)")) -> ()  [unwired: 2 in, 2 out]
          }
        }
      }
      event "BD 1 Amplitude 1 (%)", "BD 1 Amplitude 2 (%)", "BD 1 Amplitude 3 (%)", "BD 2 Amplitude 1 (%)", "BD 2 Amplitude 2 (%)", "BD 2 Amplitude 3 (%)", "Trap 1 ON", "Trap 2 ON", "Trap 3 ON", "Feedback On/Off", "All FB On/Off": Value Change {
        w1763 = i16 1 ("f")
        n521 = event-data() -> ()  [unwired: 7 out]
        n522 = local write "Trap 1 (ON/OFF)"("Trap 1 ON") -> ()
        n523 = local write "Trap 2 (ON/OFF)"("Trap 2 ON") -> ()
        n524 = Boolean To (0,1)(Boolean="Trap 3 ON") -> (0, 1=w1764:i16)
        n525 = Boolean To (0,1)(Boolean="Trap 1 ON") -> (0, 1=w1765:i16)
        n526 = Boolean To (0,1)(Boolean="Trap 2 ON") -> (0, 1=w1766:i16)
        n527 = Select(t=w1766, s="Trap ON/OFF X or Y Amp?", f=w1763) -> (s? t:f=w1761:i16)
        n528 = Select(t=w1765, s="Trap ON/OFF X or Y Amp?", f=w1763) -> (s? t:f=w1762:i16)
        n529 = Select(t=w1764, s="Trap ON/OFF X or Y Amp?", f=w1763) -> (s? t:f=w1760:i16)
        n530 = Select(t=w1763, s="Trap ON/OFF X or Y Amp?", f=w1766) -> (s? t:f=w1758:i16)
        n531 = Select(t=w1763, s="Trap ON/OFF X or Y Amp?", f=w1765) -> (s? t:f=w1759:i16)
        n532 = Select(t=w1763, s="Trap ON/OFF X or Y Amp?", f=w1764) -> (s? t:f=w1757:i16)
        n533 = And(x="All FB On/Off", y="Feedback On/Off") -> (x .and. y?=w1755:cluster{"Set 1":bool, "Set 2":bool})
        n534 = local read "BD 1 Amplitude 1 (%)"() -> (w1775:dbl)
        n535 = local read "BD 1 Amplitude 2 (%)"() -> (w1774:dbl)
        n536 = local read "BD 1 Amplitude 3 (%)"() -> (w1773:dbl)
        n537 = Unbundle By Name(w1755) -> ("Set 1"=w1750:bool, "Set 2"=w1747:bool)
        n538 = local read "Y RF Amplitude Limits (%)"() -> (w1743:T16)
        n539 = local read "X RF Amplitude Limits (%)"() -> (w1744:T16)
        n540 = local read "BD 2 Amplitude 1 (%)"() -> (w1776:dbl)
        n541 = local read "BD 2 Amplitude 2 (%)"() -> (w1777:dbl)
        n542 = local read "BD 2 Amplitude 3 (%)"() -> (w1778:dbl)
        n543 = And(x="Trap 2 ON", y=w1747) -> (x .and. y?=w1745:bool)
        n544 = And(x="Trap 1 ON", y=w1750) -> (x .and. y?=w1748:bool)
        n545 = Multiply(x=w1762, y=w1775) -> (x*y=w1770:dbl)
        n546 = Multiply(x=w1774, y=w1761) -> (x*y=w1768:dbl)
        n547 = Multiply(x=w1773, y=w1760) -> (x*y=w1769:dbl)
        n548 = Multiply(x=w1776, y=w1759) -> (x*y=w1779:dbl)
        n549 = Multiply(x=w1777, y=w1758) -> (x*y=w1780:dbl)
        n550 = Multiply(x=w1778, y=w1757) -> (x*y=w1781:dbl)
        n551 = call "set RF board amplitude - interlace.vi"("Board 2 Amplitude Limits"=w1743, "Board 1 Amplitude Limits"=w1744, "error in"=w1771, "FPGA VI Reference In"=w1772, "Board 2 Amplitude 3 (%)"=w1781, "Board 1 Amplitude 3 (%)"=w1769, "Board 2 Amplitude 2 (%)"=w1780, "Board 2 Amplitude 1 (%)"=w1779, "Board 1 Amplitude 2 (%)"=w1768, "Board 1 Amplitude 1 (%)"=w1770) -> ("error out"=w1752:errorcluster, "FPGA VI Reference Out"=w1753:T19)
        n552 = xnode "Read/Write Control"("FPGA VI Reference In"=w1753, "error in"=w1752, "FB On/Off Set 1"=w1748, "FB On/Off Set 2"=w1745) -> ("error out"=w1751:errorcluster)  [unwired: 1 out]
      }
      event "Load parameters": Value Change {
        n553 = event-data() -> ()  [unwired: 7 out]
        n554 = property on="Saved AOD Raster Scan Parameter Sets" class="Arr (strict)"() -> ("Index Values"=w1851:u32[])  [unwired: 2 in, 2 out]
        n555 = Index Array(array=w1851, index=0) -> (element=w1848:u32)
        n556 = local write "Load parameters"(FALSE ("Load parameters")) -> ()
        n557 = Index Array(array="Saved AOD Raster Scan Parameter Sets", index=w1848) -> (element=w1847:T32)
        n558 = Unbundle By Name(w1847) -> ("Scan Range AOD (nm) 2"=w1846:dbl, "Step Size AOD (nm) 2"=w1845:dbl, "Scan Speed AOD (nm/s) 2"=w1844:dbl, "Number of scans (AOD) 2"=w1843:u16)
        n559 = flat-sequence {
          tunnel: w1846 -> [w1854]
          tunnel: w1845 -> [w1853]
          tunnel: w1844 -> [w1852]
          tunnel: w1843 -> [w1855]
          frame #0 {
            n560 = local write "Scan Speed (nm/s)"(w1852) -> ()
            n561 = local write "Scan Range (nm)"(w1854) -> ()
            n562 = local write "Step Size (nm)"(w1853) -> ()
          }
          frame #1 {
            n563 = property on="Number of F/B Scans (AOD)" class="DigNum (strict)"("Val(Sgnl)"=w1855) -> ()  [unwired: 2 in, 2 out]
          }
        }
      }
      event "Trap 1 (ON/OFF)", "Trap 2 (ON/OFF)": Value Change {
        n564 = event-data() -> ()  [unwired: 7 out]
        n565 = property on="Trap 2 ON" class="Bool (strict)"("Val(Sgnl)"="Trap 2 (ON/OFF)") -> ()  [unwired: 2 in, 2 out]
        n566 = property on="Trap 1 ON" class="Bool (strict)"("Val(Sgnl)"="Trap 1 (ON/OFF)") -> ()  [unwired: 2 in, 2 out]
      }
      event "DIO count 1 (ticks)", "DIO count 2 (ticks)", "DIO count 3 (ticks)", "Interlace", "Number Interlace Sets", "Not-Interlacing Set": Value Change {
        n567 = event-data() -> ()  [unwired: 7 out]
        n568 = local read "DIO count 3 (ticks)"() -> (w1868:u32)
        n569 = local read "DIO count 1 (ticks)"() -> (w1870:u32)
        n570 = local read "DIO count 2 (ticks)"() -> (w1869:u32)
        n571 = To Unsigned Byte Integer(number="Not-Interlacing Set") -> (unsigned 8bit integer=w1859:u8)
        n572 = Add(x=w1859, y=u8 1) -> (x+y=w1863:u8)
        n573 = xnode "Read/Write Control"("FPGA VI Reference In"=w1874, "error in"=w1872, "DIO count 1 (ticks)"=w1870, "DIO count 2 (ticks)"=w1869, "DIO count 3 (ticks)"=w1868, "Interlace ON/OFF"="Interlace", "Number Interlace Cycles"="Number Interlace Sets", "Interlace Off Parameters"=w1863) -> ("error out"=w1873:errorcluster)  [unwired: 1 out]
        n574 = Build Array(w1870, w1869, w1868) -> (w1861:u32[])
        n575 = Split 1D Array(array=w1861, index="Number Interlace Sets") -> (first subarray=w1871:u32[])  [unwired: 1 out]
        n576 = Index Array(array=w1861, index=w1859) -> (element=w1860:u32)
        n577 = Add Array Elements(numeric array=w1871) -> (sum=w1865:u32)
        n578 = Select(t=w1865, s="Interlace", f=w1860) -> (s? t:f=→"Total Counts (ticks)":u32)
      }
      event "Reset Feedback": Value Change {
        n579 = event-data() -> ()  [unwired: 7 out]
        n580 = Unbundle By Name("Reset Feedback") -> ("Set 1"=w2016:bool, "Set 2"=w2015:bool)
        n581 = xnode "Read/Write Control"("FPGA VI Reference In"=w2018, "error in"=w2013, "FB Reset Set 1"=w2016, "FB Reset Set 2"=w2015) -> ("error out"=w2014:errorcluster)  [unwired: 1 out]
      }
      event "PID Gains": Value Change {
        n582 = event-data() -> ()  [unwired: 7 out]
        n583 = Unbundle By Name("PID Gains") -> ("Set 1"=w2081:T14, "Set 2"=w2080:T14)
        n584 = xnode "Read/Write Control"("FPGA VI Reference In"=w2082, "error in"=w2078, "FB Gains Set 1"=w2081, "FB Gains Set 2"=w2080) -> ("error out"=w2079:errorcluster)  [unwired: 1 out]
      }
      event "AI2 to Setpoint", "Trap Intensity\nSetpoints (V)": Value Change {
        n585 = event-data() -> ()  [unwired: 7 out]
        n586 = xnode "Read/Write Control"("FPGA VI Reference In"=w2157, "error in"=w2153) -> ("FPGA VI Reference Out"=w2156:T19, "error out"=w2155:errorcluster, "AI2 Y Sum Set 1"=w2164:i16, "AI2 Y Sum Set 2"=w2163:i16)
        n587 = Cluster To Array(cluster="AI2 to Setpoint") -> (array=w2167:bool[])
        n588 = local read "AI2 (V)"() -> (w2165:cluster{"Set 1":dbl, "Set 2":dbl})
        n589 = Or Array Elements(Boolean array=w2167) -> (logical OR=w2168:bool)
        n590 = Bundle By Name(cluster=w2165, "Set 1"=w2164, "Set 2"=w2163) -> (w2162:cluster{"Set 1":dbl, "Set 2":dbl})
        n591 = Divide(x=w2162, y=3276.7) -> (x/y=w2161:cluster{"Set 1":dbl, "Set 2":dbl})
        "AI2 (V)" <- w2161
        n592 = case shown="True" w2168 {
          tunnel: [w2232 w2249] -> w2160
          tunnel: "AI2 to Setpoint" -> [_ w2245]
          tunnel: "Trap Intensity\nSetpoints (V)" -> [w2233 w2248]
          tunnel: w2161 -> [_ w2242]
          frame False {
            n593 = Multiply(x=3276.7, y=w2233) -> (x*y=w2234:cluster{"Set 1":dbl, "Set 2":dbl})
            n594 = To Word Integer(number=w2234) -> (16bit integer=w2232:cluster{"Set 1":i16, "Set 2":i16})
          }
          frame True {
            n595 = Unbundle By Name(w2242) -> ("Set 1"=w2241:dbl, "Set 2"=w2240:dbl)
            n596 = Unbundle By Name(w2248) -> ("Set 1"=w2247:dbl, "Set 2"=w2246:dbl)
            n597 = Unbundle By Name(w2245) -> ("Set 1"=w2244:bool, "Set 2"=w2243:bool)
            n598 = Select(t=w2241, s=w2244, f=w2247) -> (s? t:f=w2239:dbl)
            n599 = Select(t=w2240, s=w2243, f=w2246) -> (s? t:f=w2238:dbl)
            n600 = Bundle By Name(cluster=w2248, "Set 1"=w2239, "Set 2"=w2238) -> (w2236:cluster{"Set 1":dbl, "Set 2":dbl})
            n601 = local write "Trap Intensity\nSetpoints (V)"(w2236) -> ()
            n602 = Multiply(x=3276.7, y=w2236) -> (x*y=w2237:cluster{"Set 1":dbl, "Set 2":dbl})
            n603 = To Word Integer(number=w2237) -> (16bit integer=w2249:cluster{"Set 1":i16, "Set 2":i16})
          }
        }
        n604 = Unbundle By Name(w2160) -> ("Set 1"=w2159:i16, "Set 2"=w2158:i16)
        n605 = xnode "Read/Write Control"("FPGA VI Reference In"=w2156, "error in"=w2155, "FB Setpoint Set 1"=w2159, "FB Setpoint Set 2"=w2158) -> ("error out"=w2154:errorcluster)  [unwired: 1 out]
      }
      event "Invert GI": Value Change {
        n606 = event-data() -> ()  [unwired: 7 out]
        n607 = xnode "Read/Write Control"("FPGA VI Reference In"=w2311, "error in"=w2309, "Invert GI"="Invert GI", "Invert GI 2"="Invert GI") -> ("error out"=w2310:errorcluster)  [unwired: 1 out]
      }
      event "Green FB Setpoint (mV)", "Green FB Gains", "Green FB On/Off", "Current When FB OFF (%)", "Green int current ON count adj": Value Change {
        n608 = event-data() -> ()  [unwired: 7 out]
        n609 = local read "Green FB Setpoint (mV)"() -> (w2377:dbl)
        n610 = local read "Current When FB OFF (%)"() -> (w2380:dbl)
        n611 = Multiply(x=w2377, y=3.2767) -> (x*y=w2376:dbl)
        n612 = Multiply(x=w2380, y=655.35) -> (x*y=w2381:dbl)
        n613 = To Unsigned Word Integer(number=w2381) -> (unsigned 16bit integer=w2379:u16)
        n614 = local read "Green int current ON count adj"() -> (w2384:u32)
        n615 = local read "Green FB Gains"() -> (w2383:T14)
        n616 = local read "Green Laser ON/Interlacing"() -> (w2374:bool)
        n617 = local read "Green laser mode"() -> (w2373:enum32{"Laser ON", "Laser OFF", "Interlace"})
        n618 = local read "Green FB On/Off"() -> (w2385:bool)
        n619 = Equal?(x=w2373, y=enum32{"Laser ON", "Laser OFF", "Interlace"}."Interlace") -> (x = y?=w2371:bool)
        n620 = Compound Arithmetic op=AND(w2371, w2385, w2374) -> (w2375:bool)
        n621 = xnode "Read/Write Control"("FPGA VI Reference In"=w2388, "error in"=w2387, "Green FB Setpoint"=w2376, "Green FB On/Off"=w2375, "Current Out"=w2379, "Green int current ON count adj"=w2384, "Green FB Gains"=w2383) -> ("error out"=w2386:errorcluster)  [unwired: 1 out]
      }
      event "Green laser mode", "Green Laser ON/Interlacing": Value Change {
        n622 = event-data() -> ()  [unwired: 7 out]
        n623 = case shown="True" "Green Laser ON/Interlacing" {
          tunnel: "Green laser mode" -> [_ w2526]
          tunnel: [enum32{"Laser ON", "Laser OFF", "Interlace"}."Laser OFF" ("Green laser mode") w2526] -> w2514
          tunnel: [FALSE w2522] -> w2513
          frame False {
          }
          frame True {
            n624 = local read "Green FB On/Off"() -> (w2523:bool)
            n625 = Equal?(x=w2526, y=enum32{"Laser ON", "Laser OFF", "Interlace"}."Interlace") -> (x = y?=w2524:bool)
            n626 = And(x=w2524, y=w2523) -> (x .and. y?=w2522:bool)
          }
        }
        n627 = xnode "Read/Write Control"("FPGA VI Reference In"=w2519, "error in"=w2517, "Operating Mode"=w2514, "Operating Mode 2"=w2514, "Green FB On/Off"=w2513) -> ("error out"=w2518:errorcluster)  [unwired: 1 out]
      }
      event "- phase (APD 1 Gate)", "+ phase (APD 1 Gate)": Value Change {
        n628 = event-data() -> ()  [unwired: 7 out]
        n629 = local read "Phase Adj. (APD 1 Gate)"() -> (w2605:i16)
        n630 = Negate(x=w2605) -> (-x=w2613:i16)
        n631 = Select(t=w2613, s="- phase (APD 1 Gate)", f=w2605) -> (s? t:f=w2612:i16)
        n632 = Or(x="- phase (APD 1 Gate)", y="+ phase (APD 1 Gate)") -> (x .or. y?=w2608:bool)
        n633 = xnode "Read/Write Control"("FPGA VI Reference In"=w2615, "error in"=w2614, "Phase count adjustment (APD 1 Gate)"=w2612) -> ("FPGA VI Reference Out"=w2610:T19, "error out"=w2611:errorcluster)
        n634 = xnode "Read/Write Control"("FPGA VI Reference In"=w2610, "error in"=w2611, "+ phase (APD 1 Gate)"=w2608) -> ("error out"=w2609:errorcluster)  [unwired: 1 out]
      }
      event "+ phase (APD 2 Gate)", "- phase (APD 2 Gate)": Value Change {
        n635 = event-data() -> ()  [unwired: 7 out]
        n636 = local read "Phase Adj. (APD 2 Gate)"() -> (w2691:i16)
        n637 = Negate(x=w2691) -> (-x=w2699:i16)
        n638 = Select(t=w2699, s="- phase (APD 2 Gate)", f=w2691) -> (s? t:f=w2698:i16)
        n639 = Or(x="- phase (APD 2 Gate)", y="+ phase (APD 2 Gate)") -> (x .or. y?=w2694:bool)
        n640 = xnode "Read/Write Control"("FPGA VI Reference In"=w2701, "error in"=w2700, "Phase count adjustment (APD 2 Gate)"=w2698) -> ("FPGA VI Reference Out"=w2696:T19, "error out"=w2697:errorcluster)
        n641 = xnode "Read/Write Control"("FPGA VI Reference In"=w2696, "error in"=w2697, "+ phase (APD 2 Gate)"=w2694) -> ("error out"=w2695:errorcluster)  [unwired: 1 out]
      }
      event "Phase Adj. (APD Acq)", "+ phase (APD Acq)", "- phase (APD Acq)": Value Change {
        n642 = event-data() -> ()  [unwired: 7 out]
        n643 = local read "Phase Adj. (APD Acq)"() -> (w2779:i16)
        n644 = Negate(x=w2779) -> (-x=w2785:i16)
        n645 = Select(t=w2785, s="+ phase (APD Acq)", f=w2779) -> (s? t:f=w2784:i16)
        n646 = Or(x="+ phase (APD Acq)", y="- phase (APD Acq)") -> (x .or. y?=w2780:bool)
        n647 = xnode "Read/Write Control"("FPGA VI Reference In"=w2787, "error in"=w2786, "Phase Count Adjustment (APD Acq)"=w2784) -> ("FPGA VI Reference Out"=w2782:T19, "error out"=w2783:errorcluster)
        n648 = xnode "Read/Write Control"("FPGA VI Reference In"=w2782, "error in"=w2783, "+ phase (APD Acq)"=w2780) -> ("error out"=w2781:errorcluster)  [unwired: 1 out]
      }
      event "Phase adj. (GI)", "+ phase (GI)", "- phase (GI)": Value Change {
        n649 = event-data() -> ()  [unwired: 7 out]
        n650 = Negate(x="Phase adj. (GI)") -> (-x=w2871:i16)
        n651 = Select(t=w2871, s="+ phase (GI)", f="Phase adj. (GI)") -> (s? t:f=w2870:i16)
        n652 = Or(x="+ phase (GI)", y="- phase (GI)") -> (x .or. y?=w2866:bool)
        n653 = xnode "Read/Write Control"("FPGA VI Reference In"=w2873, "error in"=w2872, "Phase count adjustment (GI)"=w2870) -> ("FPGA VI Reference Out"=w2868:T19, "error out"=w2869:errorcluster)
        n654 = xnode "Read/Write Control"("FPGA VI Reference In"=w2868, "error in"=w2869, "+ phase (GI)"=w2866) -> ("error out"=w2867:errorcluster)  [unwired: 1 out]
      }
      event "Phase adj. (GI) 2", "+ phase (GI) 2", "- phase (GI) 2": Value Change {
        n655 = event-data() -> ()  [unwired: 7 out]
        n656 = Negate(x="Phase adj. (GI) 2") -> (-x=w2957:i16)
        n657 = Select(t=w2957, s="+ phase (GI) 2", f="Phase adj. (GI) 2") -> (s? t:f=w2956:i16)
        n658 = Or(x="+ phase (GI) 2", y="- phase (GI) 2") -> (x .or. y?=w2952:bool)
        n659 = xnode "Read/Write Control"("FPGA VI Reference In"=w2959, "error in"=w2958, "Phase count adjustment (GI) 2"=w2956) -> ("FPGA VI Reference Out"=w2954:T19, "error out"=w2955:errorcluster)
        n660 = xnode "Read/Write Control"("FPGA VI Reference In"=w2954, "error in"=w2955, "+ phase (GI) 2"=w2952) -> ("error out"=w2953:errorcluster)  [unwired: 1 out]
      }
      event "Phase adj. (Green FB)", "- phase (Green FB)", "+ phase (Green FB)": Value Change {
        n661 = event-data() -> ()  [unwired: 7 out]
        n662 = Negate(x="Phase adj. (Green FB)") -> (-x=w3043:i16)
        n663 = Select(t=w3043, s="+ phase (Green FB)", f="Phase adj. (Green FB)") -> (s? t:f=w3042:i16)
        n664 = Or(x="+ phase (Green FB)", y="- phase (Green FB)") -> (x .or. y?=w3038:bool)
        n665 = xnode "Read/Write Control"("FPGA VI Reference In"=w3045, "error in"=w3044, "Phase count adjustment (Green FB)"=w3042) -> ("FPGA VI Reference Out"=w3040:T19, "error out"=w3041:errorcluster)
        n666 = xnode "Read/Write Control"("FPGA VI Reference In"=w3040, "error in"=w3041, "+ phase (Green FB)"=w3038) -> ("error out"=w3039:errorcluster)  [unwired: 1 out]
      }
      event "Invert APD Gate", "APD Gate ON Count", "APD Gate OFF Count", "APD Gate", "APD Integration Time (s)", "APD 1 AO Mult.", "APD 2 AO Mult.": Value Change {
        n667 = event-data() -> ()  [unwired: 7 out]
        n668 = local read "APD Integration Time (s)"() -> (w3121:dbl)
        n669 = local read "APD Gate ON Count"() -> (w3134:u32)
        n670 = local read "APD Gate OFF Count"() -> (w3133:u32)
        n671 = local read "Invert APD Gate"() -> (w3135:bool)
        n672 = local read "APD Gate"() -> (w3132:enum32{"ON", "OFF", "Interlace"})
        n673 = Multiply(x=w3121, y=40000000.0) -> (x*y=w3130:dbl)
        n674 = Reciprocal(x=w3121) -> (1/x=→"APD Acq Rate (Hz)":dbl)
        n675 = To Unsigned Long Integer(number=w3130) -> (unsigned 32bit integer=w3129:u32)
        n676 = local read "DMA Update Period (s)"() -> (w3122:dbl)
        n677 = Divide(x=w3122, y=w3121) -> (x/y=w3125:dbl)
        n678 = local read "APD 1 AO Mult."() -> (w3127:i16)
        n679 = local read "APD 2 AO Mult."() -> (w3126:i16)
        n680 = Multiply(x=2.0, y=w3125) -> (x*y=w3124:dbl)
        n681 = local write "APD Samples/FIFO Acq."(w3125) -> ()
        n682 = local write "APD Elements/DMA read"(w3124) -> ()
        n683 = xnode "Read/Write Control"("FPGA VI Reference In"=w3138, "error in"=w3137, "Invert APD Gate"=w3135, "APD Gate ON Count"=w3134, "APD Gate OFF Count"=w3133, "APD Acq Rate Count"=w3129, "APD Gate Operating Mode"=w3132, "APD 1 AO scale factor"=w3127, "APD 2 AO scale factor"=w3126) -> ("error out"=w3136:errorcluster)  [unwired: 1 out]
      }
      event "GI Frequency, ON count", "Green FB Count", "GI Frequency, OFF count": Value Change {
        n684 = event-data() -> ()  [unwired: 7 out]
        n685 = xnode "Read/Write Control"("FPGA VI Reference In"=w3302, "error in"=w3300, "Green interlace ON count"="GI Frequency, ON count", "Green interlace OFF count"="GI Frequency, OFF count", "Green interlace ON count 2"="GI Frequency, ON count", "Green interlace OFF count 2"="GI Frequency, OFF count", "Green FB Count"="Green FB Count") -> ("error out"=w3301:errorcluster)  [unwired: 1 out]
      }
      event "Number of F/B Scans (AOD)", "Scan Speed (nm/s)", "Scan BD", "Initial delta (MHz)", "Step Size (nm)", "Scan Range (nm)": Value Change {
        w3481 = 123.0  # AOM cal (nm/MHz)
        n686 = event-data() -> ()  [unwired: 7 out]
        n687 = local read "BD 1 Frequency 1 (MHz)"() -> (w3464:dbl)
        n688 = local read "AOM X Cal (nm/MHz)"() -> (w3456:dbl)